vi "HeartBeatDetectOffline2BreathingSpectra.vi"() -> ()   [LabVIEW 2014, in "Phonocardiography.lvlib"]
uses:
  Phonocardiography.lvlib
  <vilib>/Waveform/WDTOps.llb/WDT Index Channel DBL.vi
  <vilib>/Waveform/WDTOps.llb/WDT Get Waveform Time Array DBL.vi
  <vilib>/measure/NI_MABase.lvlib
  <vilib>/gmath/NI_Gmath.lvlib
panel:
  out "RR intervals spectra avg":T1(graph)
  in  "Length [s]":dbl=120.0
  in  "Input files":path[](array[path])=[path "C:/Users/Tamas/Documents/Projektek/Szívhang/Felvételek cikkhez/breath_3_1.wav", path "C:/Users/Tamas/Documents/Projektek/Szívhang/Felvételek cikkhez/breath_3_2.wav", path "C:/Users/Tamas/Documents/Projektek/Szívhang/Felvételek cikkhez/breath_3_3.wav", path "C:/Users/Tamas/Documents/Projektek/Szívhang/Felvételek cikkhez/breath_3_4.wav", path "C:/Users/Tamas/Documents/Projektek/Szívhang/Felvételek cikkhez/breath_3_5.wav"]
  out "RR intervals Spectra":T2(graph)
  in  "Remove\nEctopic Beats":bool=TRUE
  out "pNN50 [%]":dbl=21.232876712328768 format="%.1f"
  out "rMSSD  [ms] 2":dbl=68.85967760569123
  out "sdRR [ms]":dbl=81.8447364744125
  out "Mean RR [ms]":dbl=843.4299467994049 format="%_1f"
  out "Mean heart rate [BPM]":dbl=71.13809537790807 format="%#.1g"
  in  "Negate":bool
  out "Heart rate":T3(graph)=[{"X [s]"=[1.0717460317460312, 1.80517006802721, 2.5313378684807244, 3.290975056689341, 4.021224489795917, 4.70439909297052, 5.478639455782311, 6.424126984126981, 7.393197278911561, 7.796190476190473, 8.327437641723353, 8.847437641723353, 9.405170068027207, 9.964353741496595, 10.772154195011334, 11.603537414965981, 12.395011337868475, 13.184852607709745, 14.145306122448973, 15.155192743764166, 16.14068027210884, 17.033469387755094, 17.822131519274368, 18.64335600907029, 19.487619047619038, 20.375328798185933, 21.22839002267573, 22.09015873015872, 23.05795918367346, 24.05832199546484, 24.99410430839001, 25.799637188208607, 26.6073469387755, 27.47473922902493, 28.39437641723355, 29.231383219954637, 29.97877551020407, 30.762539682539668, 31.684172335600895, 32.67800453514738, 33.57396825396824, 34.4517006802721, 35.36925170068026, 36.28861678004534, 37.15555555555554, 37.95655328798184, 38.77551020408161, 39.65396825396824, 40.55764172335599, 41.41306122448978, 42.231564625850325, 43.0978684807256, 43.9931065759637, 44.85678004535146, 45.67555555555553, 46.53306122448978, 47.4449886621315, 48.34476190476188, 49.17569160997731, 49.996462585033996, 50.84081632653059, 51.72117913832197, 52.59909297052152, 53.41514739229023, 54.19619047619045, 55.033197278911544, 55.98503401360542, 56.90684807256233, 57.75981859410428, 58.61931972789113, 59.50086167800451, 60.36961451247163, 61.17061224489793, 61.92444444444442, 62.72108843537412, 63.64117913832197, 64.58993197278909, 65.45814058956913, 66.26476190476188, 67.12761904761902, 67.99945578231289, 68.84235827664396, 69.60662131519271, 70.34802721088433, 71.14340136054419, 72.01424036281176, 72.89895691609975, 73.7321541950113, 74.63265306122446, 75.49950113378682, 76.35229024943307, 77.16163265306119, 77.9244444444444, 78.7406802721088, 79.62376417233557, 80.51482993197276, 81.34285714285711, 82.16371882086165, 82.98585034013603, 83.80099773242627, 84.58294784580495, 85.30902494331062, 86.04371882086164, 86.8790929705215, 87.71265306122446, 88.51310657596368, 89.29442176870745, 90.11845804988658, 91.04770975056685, 91.951746031746, 92.83129251700676, 93.60943310657592, 94.33342403628114, 95.11464852607706, 96.10811791383216, 97.0424489795918, 97.87301587301583, 98.73560090702944, 99.6119727891156, 100.47990929705212, 101.28988662131515, 102.05941043083895, 102.92235827664395, 103.86539682539679, 104.79102040816322, 105.62947845804985, 106.49442176870744, 107.41741496598635, 108.33024943310653, 109.14539682539677, 109.91655328798181, 110.7006802721088, 111.55909297052149, 112.48725623582762, 113.36698412698408, 114.20988662131515, 115.1309750566893, 116.04380952380947, 116.96145124716548, 117.8107936507936, 118.61242630385482, 119.44879818594099, 120.3123809523809, 121.14938775510198, 121.9503854875283, 122.88353741496593, 123.8236734693877], "Heart Rate [BPM]"=[70.17078604009762, 81.80806331931737, 82.62553085186114, 78.98507462686567, 82.1637063718793, 87.82527881040896, 77.49531396438616, 63.4593246354567, 61.9150131037065, 76.9022492495641, 112.94177906778204, 115.38461538461549, 107.57846804358446, 107.2992700729927, 74.27576914439706, 72.16888500981902, 75.80793032317217, 75.96463022508034, 62.47048824251586, 59.41261002335189, 60.88357109986189, 67.20512039012517, 76.07820586543993, 73.06163021868771, 71.06789858186532, 67.5896597527331, 70.33492822966507, 69.62425007893924, 61.996251171508796, 59.978239187596536, 64.11747601046817, 74.48485530908663, 74.28411005053344, 69.17285370699592, 65.24312062333553, 71.68400520156047, 80.27912621359225, 76.55363962504369, 65.1018600531442, 60.37236469836633, 66.96699736788844, 68.35796217836082, 65.39145907473319, 65.26243093922655, 69.20903954802297, 74.90657909636512, 73.26392734522106, 68.30149716055729, 66.39566395663958, 70.14102428162433, 73.30452127659571, 69.25976337556331, 67.02127659574438, 69.4706994328922, 73.28015952143613, 69.97038290670581, 65.79470857370208, 66.6834677419358, 72.20827420587224, 73.10200022101891, 71.06026426039328, 68.15371934885671, 68.34383717326173, 73.5245081693894, 76.82034606898198, 71.68400520156017, 63.03602058319041, 65.08904850929875, 70.34240748617624, 69.80793583790614, 68.0625578763246, 69.06452286489902, 74.90657909636512, 79.59331007099007, 75.31595126949817, 65.21096214511041, 63.240917782026656, 69.10781445883887, 74.38434723940055, 69.53642384106003, 68.82022471910156, 71.18261056709309, 78.50700213624546, 80.92733056031278, 75.43619568936026, 68.89907301322785, 67.81833094115196, 72.01175702155534, 66.62973408541474, 69.21628125980924, 70.35737077217718, 74.13425977810115, 78.65636147443578, 73.50816757417483, 67.94371405094435, 67.33509771986985, 72.46138678935228, 73.09392265193387, 72.98102383053818, 73.60632024034778, 76.73123767544372, 82.63585259213028, 81.66666666666627, 71.82410423452838, 71.98041349292603, 74.95750708215405, 76.7935918272568, 72.81232801320907, 64.5680819912155, 66.36901775860288, 68.21697432195603, 77.10688891479184, 82.87396642445408, 76.80250783699069, 60.39441248972906, 64.21706630424238, 72.23981653379944, 69.5583596214511, 68.46408611053663, 69.12948061448333, 74.07614781635012, 77.97029702970353, 69.5291149884375, 63.62412234298329, 64.82116609505185, 71.55993076590184, 69.36870805369146, 65.00589622641498, 65.72933227345021, 73.60632024034778, 77.80522230063454, 76.5182186234817, 69.8964497041425, 64.64379947229533, 68.20290751623874, 71.18261056709309, 65.14032496307271, 65.72933227345021, 65.38499555204083, 70.64288765484868, 74.84725050916548, 71.73842316451567, 69.47799600882185, 71.68400520156138, 74.90657909636447, 64.29821150855413, 63.82054992764095]}, {"X [s]"=array[1368064 elements], "Heart Rate [BPM]"=array[1368064 elements]}]
  out "Heart beats":cluster{"Peaks X":dbl[], "Peaks Y":dbl[]}[](graph)=[{"Peaks X"=array[1368064 elements], "Peaks Y"=array[1368064 elements]}, {"Peaks X"=[0.21668934240362803, 1.0717460317460312, 1.80517006802721, 2.5313378684807244, 3.290975056689341, 4.021224489795917, 4.70439909297052, 5.478639455782311, 6.424126984126981, 7.393197278911561, 7.796190476190473, 8.327437641723353, 8.847437641723353, 9.405170068027207, 9.964353741496595, 10.772154195011334, 11.603537414965981, 12.395011337868475, 13.184852607709745, 14.145306122448973, 15.155192743764166, 16.14068027210884, 17.033469387755094, 17.822131519274368, 18.64335600907029, 19.487619047619038, 20.375328798185933, 21.22839002267573, 22.09015873015872, 23.05795918367346, 24.05832199546484, 24.99410430839001, 25.799637188208607, 26.6073469387755, 27.47473922902493, 28.39437641723355, 29.231383219954637, 29.97877551020407, 30.762539682539668, 31.684172335600895, 32.67800453514738, 33.57396825396824, 34.4517006802721, 35.36925170068026, 36.28861678004534, 37.15555555555554, 37.95655328798184, 38.77551020408161, 39.65396825396824, 40.55764172335599, 41.41306122448978, 42.231564625850325, 43.0978684807256, 43.9931065759637, 44.85678004535146, 45.67555555555553, 46.53306122448978, 47.4449886621315, 48.34476190476188, 49.17569160997731, 49.996462585033996, 50.84081632653059, 51.72117913832197, 52.59909297052152, 53.41514739229023, 54.19619047619045, 55.033197278911544, 55.98503401360542, 56.90684807256233, 57.75981859410428, 58.61931972789113, 59.50086167800451, 60.36961451247163, 61.17061224489793, 61.92444444444442, 62.72108843537412, 63.64117913832197, 64.58993197278909, 65.45814058956913, 66.26476190476188, 67.12761904761902, 67.99945578231289, 68.84235827664396, 69.60662131519271, 70.34802721088433, 71.14340136054419, 72.01424036281176, 72.89895691609975, 73.7321541950113, 74.63265306122446, 75.49950113378682, 76.35229024943307, 77.16163265306119, 77.9244444444444, 78.7406802721088, 79.62376417233557, 80.51482993197276, 81.34285714285711, 82.16371882086165, 82.98585034013603, 83.80099773242627, 84.58294784580495, 85.30902494331062, 86.04371882086164, 86.8790929705215, 87.71265306122446, 88.51310657596368, 89.29442176870745, 90.11845804988658, 91.04770975056685, 91.951746031746, 92.83129251700676, 93.60943310657592, 94.33342403628114, 95.11464852607706, 96.10811791383216, 97.0424489795918, 97.87301587301583, 98.73560090702944, 99.6119727891156, 100.47990929705212, 101.28988662131515, 102.05941043083895, 102.92235827664395, 103.86539682539679, 104.79102040816322, 105.62947845804985, 106.49442176870744, 107.41741496598635, 108.33024943310653, 109.14539682539677, 109.91655328798181, 110.7006802721088, 111.55909297052149, 112.48725623582762, 113.36698412698408, 114.20988662131515, 115.1309750566893, 116.04380952380947, 116.96145124716548, 117.8107936507936, 118.61242630385482, 119.44879818594099, 120.3123809523809, 121.14938775510198, 121.9503854875283, 122.88353741496593, 123.8236734693877], "Peaks Y"=[0.201629638671875, 0.192962646484375, 0.213836669921875, 0.209014892578125, 0.205413818359375, 0.18658447265625, 0.20831298828125, 0.272430419921875, 0.238372802734375, 0.219329833984375, 0.125732421875, 0.18994140625, 0.128082275390625, 0.09893798828125, 0.183624267578125, 0.169097900390625, 0.19970703125, 0.200042724609375, 0.220733642578125, 0.21014404296875, 0.22100830078125, 0.17681884765625, 0.207855224609375, 0.21734619140625, 0.164459228515625, 0.166290283203125, 0.189208984375, 0.193267822265625, 0.1942138671875, 0.163330078125, 0.218475341796875, 0.165557861328125, 0.157012939453125, 0.152130126953125, 0.137481689453125, 0.184234619140625, 0.1441650390625, 0.166717529296875, 0.128570556640625, 0.168548583984375, 0.168731689453125, 0.149444580078125, 0.14691162109375, 0.1910400390625, 0.15167236328125, 0.13525390625, 0.175018310546875, 0.123992919921875, 0.168548583984375, 0.15008544921875, 0.141387939453125, 0.139434814453125, 0.14385986328125, 0.151214599609375, 0.151275634765625, 0.166107177734375, 0.11834716796875, 0.174407958984375, 0.137786865234375, 0.151580810546875, 0.13751220703125, 0.139801025390625, 0.17926025390625, 0.14227294921875, 0.141571044921875, 0.14837646484375, 0.13397216796875, 0.186920166015625, 0.125518798828125, 0.149078369140625, 0.15155029296875, 0.15460205078125, 0.1619873046875, 0.116912841796875, 0.1724853515625, 0.12261962890625, 0.166290283203125, 0.150177001953125, 0.148468017578125, 0.18017578125, 0.120941162109375, 0.151336669921875, 0.158203125, 0.1790771484375, 0.137786865234375, 0.156158447265625, 0.166778564453125, 0.147857666015625, 0.17822265625, 0.1409912109375, 0.143402099609375, 0.159912109375, 0.14312744140625, 0.17120361328125, 0.1217041015625, 0.15777587890625, 0.148040771484375, 0.17626953125, 0.146087646484375, 0.119842529296875, 0.1455078125, 0.134796142578125, 0.153167724609375, 0.155242919921875, 0.149688720703125, 0.152496337890625, 0.16204833984375, 0.188507080078125, 0.146392822265625, 0.1685791015625, 0.17132568359375, 0.12103271484375, 0.1685791015625, 0.154754638671875, 0.14630126953125, 0.1690673828125, 0.1383056640625, 0.16705322265625, 0.126739501953125, 0.16619873046875, 0.13958740234375, 0.1534423828125, 0.144744873046875, 0.1336669921875, 0.157562255859375, 0.1373291015625, 0.16473388671875, 0.1514892578125, 0.15313720703125, 0.13812255859375, 0.1527099609375, 0.17401123046875, 0.150604248046875, 0.1429443359375, 0.15435791015625, 0.147735595703125, 0.1685791015625, 0.146759033203125, 0.157257080078125, 0.150054931640625, 0.152862548828125, 0.13958740234375, 0.13262939453125, 0.1474609375, 0.147857666015625, 0.157257080078125, 0.140716552734375, 0.164642333984375]}]
  in  "Max time to peak\nfrom threshold (ms)":dbl=150.0
  in  "Threshold mult 2":dbl=0.4 min=-1.0 max=1.0 step=0.05
  in  "Min time between\nbeats (ms)":dbl=450.0
  in  "width (threshold) 2":i32=3
  in  "Breathing freq \n[1/min]":dbl=15.0
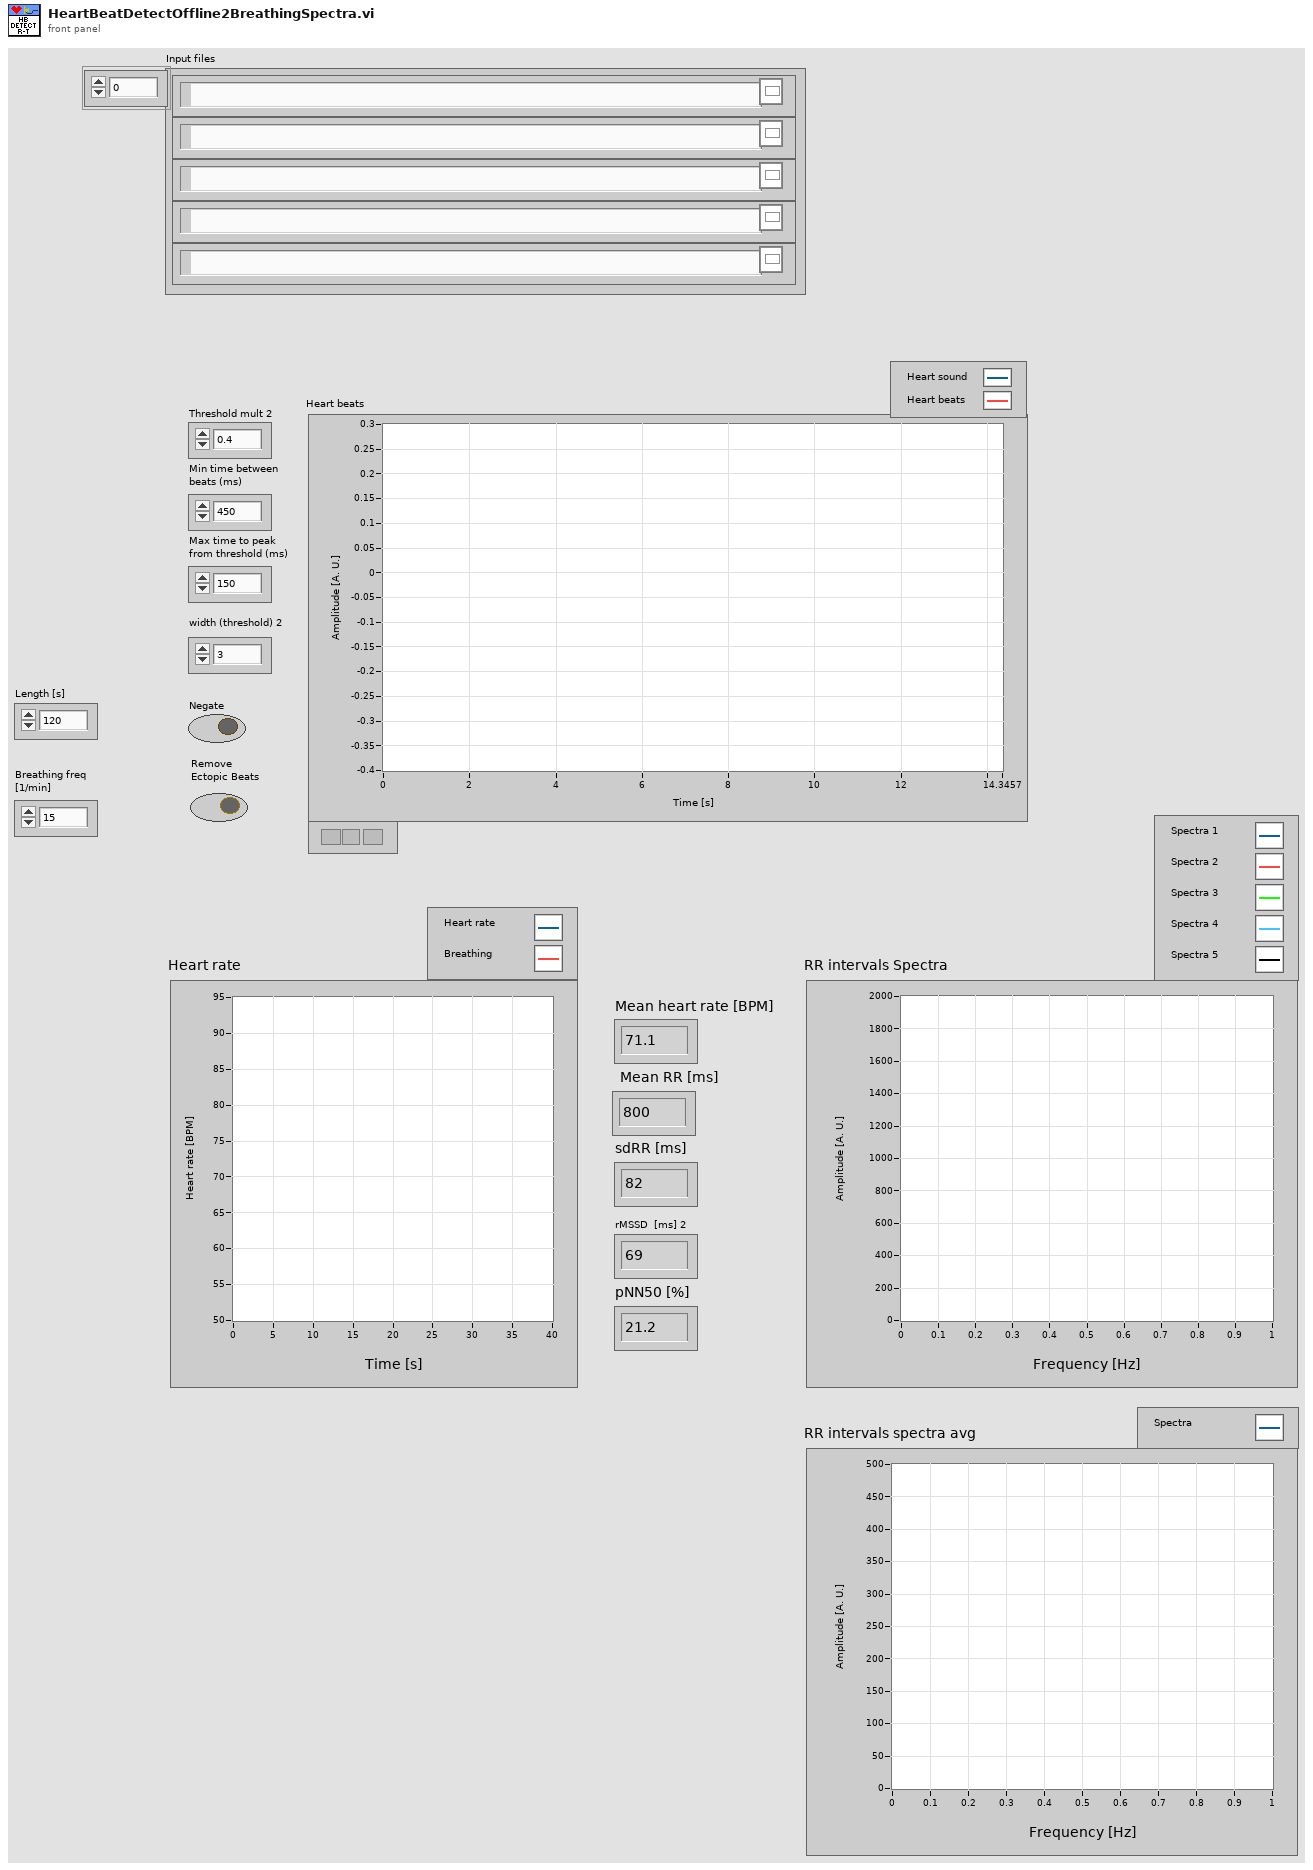
[diagram p1: front panel]
types:
  T1 = cluster{"Power Spectrum FFT {X} Frequency":dbl[], dbl[]}
  T2 = cluster{"Power Spectrum FFT {X} Frequency":dbl[], "Power Spectrum FFT {X}":dbl[]}[]
  T3 = cluster{"X [s]":dbl[], "Heart Rate [BPM]":dbl[]}[]
  T4 = typedef "LVCursorListTypeDef.ctl" = cluster{"Name":string, "Color":u32, "Style":u8, "Point Style":u8, "Name Visible":bool, "Allow Drag":bool, "Cursor Mode":u32, "Plot":i32, "Index":i32, "Position":cluster{"X":dbl, "Y":dbl}, "X Scale":u32, "Y Scale":u32, "Watch Plots":i32[], "Watch All Plots":bool, "Plot Area":i32, "Label Offset":cluster{"X":dbl, "Y":dbl}}[]
  T5 = cluster{"Name":string, "Color":u32, "Style":u8, "Point Style":u8, "Name Visible":bool, "Allow Drag":bool, "Cursor Mode":u32, "Plot":i32, "Index":i32, "Position":cluster{"X":dbl, "Y":dbl}, "X Scale":u32, "Y Scale":u32, "Watch Plots":i32[], "Watch All Plots":bool, "Plot Area":i32, "Label Offset":cluster{"X":dbl, "Y":dbl}}
  T6 = cluster{"Name":string, "Color":u32, "Style":u8, "Point Style":u8, "Name Visible":bool, "Allow Drag":bool, "Cursor Mode":u32, "Plot":i32, "Index":i32, "Position":cluster{"X":dbl, "Y":dbl}, "X Scale":u32, "Y Scale":u32, "Watch Plots":i32[], "Watch All Plots":bool, "Plot Area":i32, "Label Offset":cluster{"X":dbl, "Y":dbl}}[]
  T7 = cluster{"Power Spectrum FFT {X} Frequency":dbl[], "Power Spectrum FFT {X}":dbl[]}
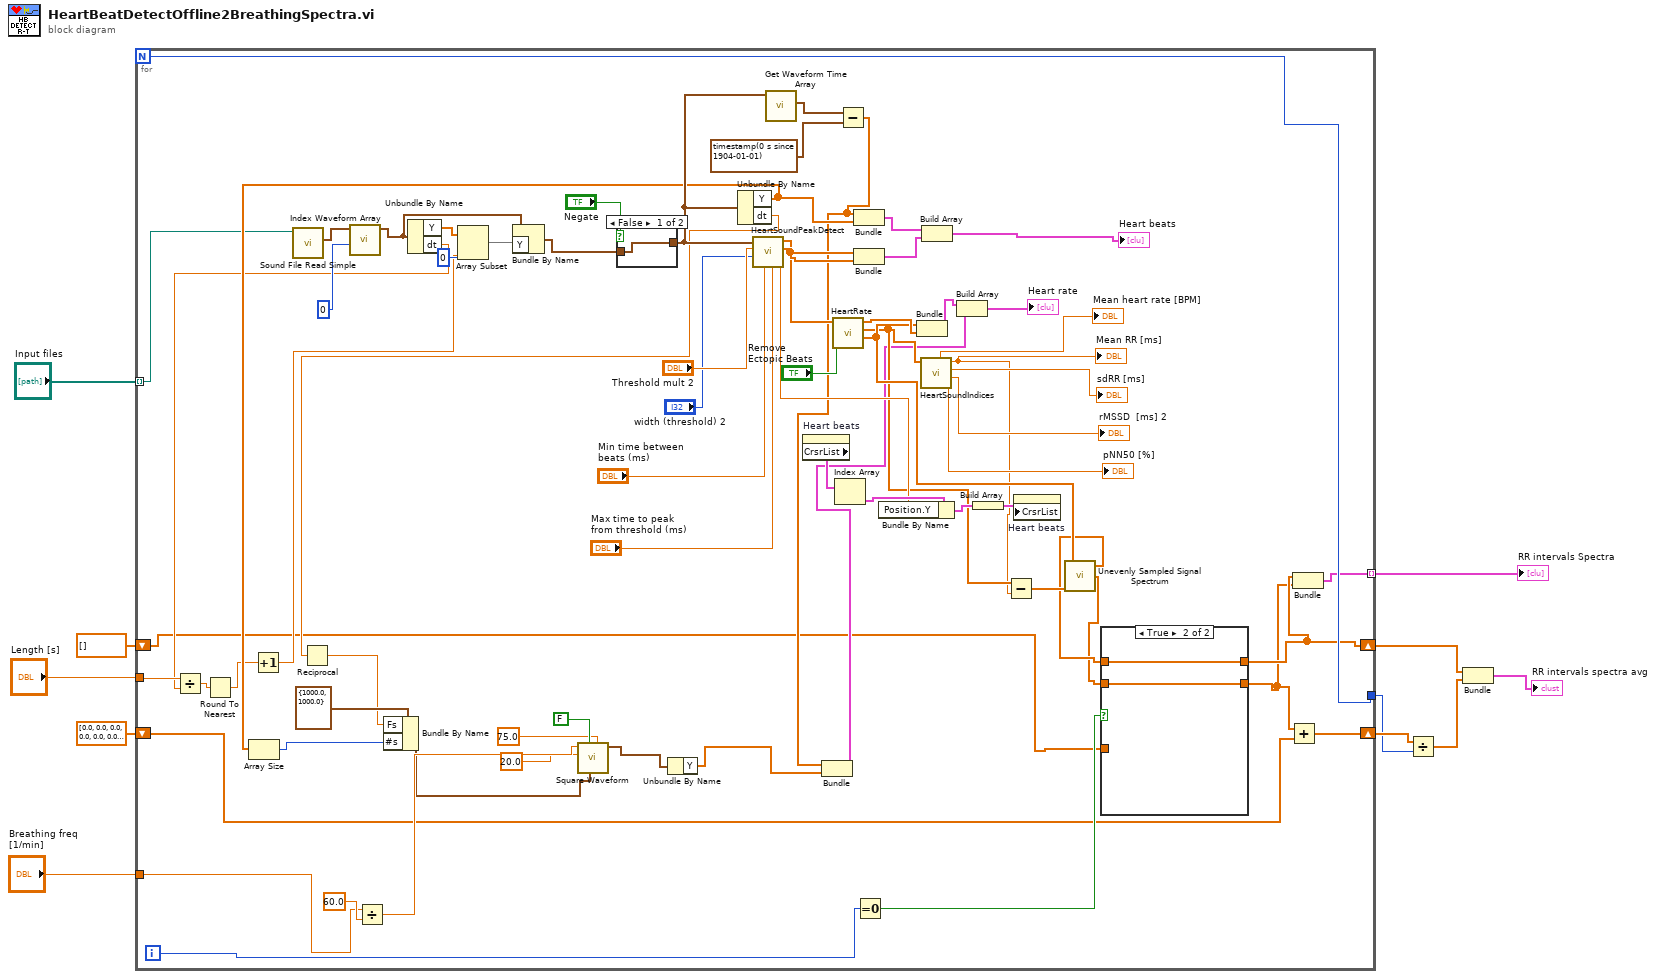
[diagram p0: block diagram]
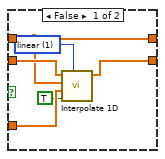
[diagram p2: hidden frame]
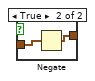
[diagram p3: hidden frame]
diagram:
  n1 = for {
    N -> [w16]
    tunnel: "Breathing freq \n[1/min]" -> [w77]
    tunnel: "Input files" -> [w34] mode=indexing
    tunnel: "Length [s]" -> [w33]
    shift-right: [w15] -> w3
    shift-left: dbl[] [] ("Power Spectrum FFT {X} Frequency") -> [w18]
    shift-right: [w17] -> w6
    shift-left: dbl[] [0.0, 0.0, 0.0, 0.0, 0.0, 0.0, 0.0, 0.0, 0.0, 0.0, 0.0, 0.0, 0.0, 0.0, 0.0, 0.0, 0.0, 0.0, 0.0, 0.0, 0.0, 0.0, 0.0, 0.0, 0.0, 0.0, 0.0, 0.0, 0.0, 0.0, 0.0, 0.0, 0.0, 0.0, 0.0, 0.0, 0.0, 0.0, 0.0, 0.0, 0.0, 0.0, 0.0, 0.0, 0.0, 0.0, 0.0, 0.0, 0.0, 0.0, 0.0, 0.0, 0.0, 0.0, 0.0, 0.0, 0.0, 0.0, 0.0, 0.0, 0.0, 0.0, 0.0, 0.0, 0.0, 0.0, 0.0, 0.0, 0.0, 0.0, 0.0, 0.0, 0.0, 0.0, 0.0, 0.0, 0.0, 0.0, 0.0, 0.0, 0.0, 0.0, 0.0, 0.0, 0.0, 0.0, 0.0, 0.0, 0.0, 0.0, 0.0, 0.0, 0.0, 0.0, 0.0, 0.0, 0.0, 0.0, 0.0, 0.0, 0.0, 0.0, 0.0, 0.0, 0.0, 0.0, 0.0, 0.0, 0.0, 0.0, 0.0, 0.0, 0.0, 0.0, 0.0, 0.0, 0.0, 0.0, 0.0, 0.0, 0.0, 0.0, 0.0, 0.0, 0.0, 0.0, 0.0, 0.0, 0.0, 0.0, 0.0, 0.0, 0.0, 0.0, 0.0, 0.0, 0.0, 0.0, 0.0, 0.0, 0.0, 0.0, 0.0, 0.0, 0.0, 0.0, 0.0, 0.0, 0.0, 0.0, 0.0] -> [w12]
    tunnel: [w16] -> w5
    tunnel: [w14] -> w4 mode=indexing
    i -> [w20]
    n2 = call <vilib>:"Sound File Read Simple.vi"("path"=w34) -> ("data"=w76:waveform(dbl)[])  [unwired: 7 in, 3 out]
    n3 = call-poly <vilib>:"Index Waveform Array.vi"("index"=0, "waveform array"=w76) -> ("waveform"=w28:waveform(dbl))  [unwired: 8 in, 1 out]
    n4 = Divide(x=w77, y=60.0) -> (x/y=w80:dbl)
    n5 = Unbundle By Name(w28) -> ("Y"=w27:dbl[], "dt"=w29:dbl)
    n6 = Divide(x=w33, y=w29) -> (x/y=w31:dbl)
    n7 = Round To Nearest(number=w31) -> (nearest integer value=w30:dbl)
    n8 = Increment(x=w30) -> (x+1=w23:dbl)
    n9 = Array Subset(array=w27, index=0, length=w23) -> (w26:dbl[])
    n10 = Bundle By Name(cluster=w28, "Y"=w26) -> (w25:waveform(dbl))
    n11 = case shown="False" "Negate" {
      tunnel: w25 -> [w90 w92]
      tunnel: [w90 w91] -> w57
      frame False {
      }
      frame True {
        n12 = Negate(x=w92) -> (-x=w91:waveform(dbl))
      }
    }
    n13 = Unbundle By Name(w57) -> ("Y"=w43:dbl[], "dt"=w32:dbl)
    n14 = Array Size(array=w43) -> (size(s)=w42:i32)
    n15 = Reciprocal(x=w32) -> (1/x=w37:dbl)
    n16 = Bundle By Name(cluster=cluster{"Fs":dbl, "#s":dbl} {"Fs"=1000.0, "#s"=1000.0} ("sampling info"), "Fs"=w37, "#s"=w42) -> (w78:cluster{"Fs":dbl, "#s":dbl})
    n17 = call <vilib>:"Square Waveform.vi"("offset"=75.0 ("amplitude"), "sampling info"=w78, "reset signal"=FALSE, "amplitude"=20.0, "frequency"=w80) -> ("signal out"=w45:waveform(dbl))  [unwired: 5 in, 1 out]
    n18 = Unbundle By Name(w45) -> ("Y"=w36:dbl[])
    n19 = call "HeartSoundPeakDetect.vi"("Max time to peak\nfrom threshold (ms)"="Max time to peak\nfrom threshold (ms)", "Min time between\nbeats (ms)"="Min time between\nbeats (ms)", "width (threshold)"="width (threshold) 2", "Threshold multiplier"="Threshold mult 2", "Sound"=w57) -> ("Threshold"=w58:dbl, "Peaks Y"=w70:dbl[], "Peaks X"=w67:dbl[])  [unwired: 4 in]
    n20 = call-poly <vilib>:"Get Waveform Time Array.vi"("waveform in"=w57) -> ("X array"=w65:timestamp[])  [unwired: 9 in, 1 out]
    n21 = property on="Heart beats" class="XYGraph (strict)"() -> ("CrsrList"=w60:T4)  [unwired: 2 in, 2 out]
    n22 = call "HeartRate.vi"("Remove Ectopic?"="Remove\nEctopic Beats", "Peaks X in"=w67) -> ("X [s]"=w50:dbl[], "RR intervals [ms]"=w48:dbl[], "Heart Rate [BPM]"=w66:dbl[])  [unwired: 7 in]
    n23 = Index Array(array=w60) -> (element=w62:T5)  [unwired: 1 in]
    n24 = Subtract(x=w65, y=timestamp(0 s since 1904-01-01) ("Xo")) -> (x-y=w41:dbl[])
    n25 = Bundle(w41, "Y"=w36) -> (w39:cluster{dbl[], "Y":dbl[]})  [unwired: 1 in]
    n26 = Bundle(w41, "Y"=w43) -> (w69:cluster{dbl[], "Y":dbl[]})  [unwired: 1 in]
    n27 = Bundle("Peaks X"=w67, "Peaks Y"=w70) -> (w68:cluster{"Peaks X":dbl[], "Peaks Y":dbl[]})  [unwired: 1 in]
    n28 = Equal To 0?(x=w20) -> (x = 0?=w19:bool)
    n29 = Bundle By Name(cluster=w62, "Position.Y"=w58) -> (w61:T5)
    n30 = Bundle("X [s]"=w50, "Heart Rate [BPM]"=w66) -> (w40:cluster{"X [s]":dbl[], "Heart Rate [BPM]":dbl[]})  [unwired: 1 in]
    n31 = call "HeartSoundIndices.vi"("RR intervals [ms]"=w48) -> ("pNN50 [%]"=→"pNN50 [%]":dbl, "rMSSD  [ms]"=→"rMSSD  [ms] 2":dbl, "sdRR [ms]"=→"sdRR [ms]":dbl, "Mean RR [ms]"=w47:dbl, "Mean heart rate [BPM]"=→"Mean heart rate [BPM]":dbl)  [unwired: 6 in]
    "Mean RR [ms]" <- w47
    n32 = Build Array(w69, w68) -> (→"Heart beats":cluster{"Peaks X":dbl[], "Peaks Y":dbl[]}[])
    n33 = Build Array(w40, w39) -> (→"Heart rate":cluster{"X [s]":dbl[], "Y":dbl[]}[])
    n34 = Build Array(w61) -> (w59:T6)
    n35 = Subtract(x=w48, y=w47) -> (x-y=w49:dbl[])
    n36 = property on="Heart beats" class="XYGraph (strict)"("CrsrList"=w59) -> ()  [unwired: 2 in, 2 out]
    n37 = call <vilib>:"Unevenly Sampled Signal Spectrum.vi"("XTime"=w50, "X"=w49) -> ("Power Spectrum FFT {X} Frequency"=w22:dbl[], "Power Spectrum FFT {X}"=w21:dbl[])  [unwired: 1 out]
    n38 = case shown="True" w19 {
      tunnel: w22 -> [w86 w89]
      tunnel: w21 -> [w87 w88]
      tunnel: [w86 w89] -> w15
      tunnel: [w83 w88] -> w13
      tunnel: w18 -> [w85 _]
      frame False {
        w82 = 1 items=["nearest", "linear", "spline", "cubic Hermite", "Lagrange"] ("method")
        n39 = call <vilib>:"Interpolate 1D.vi"("method"=w82, "X is monotonic"=TRUE, "xi"=w85, "X"=w86, "Y"=w87) -> ("yi"=w83:dbl[])  [unwired: 4 in, 2 out]
      }
      frame True {
      }
    }
    n40 = Add(x=w13, y=w12) -> (x+y=w17:dbl[])
    n41 = Bundle("Power Spectrum FFT {X} Frequency"=w15, "Power Spectrum FFT {X}"=w13) -> (w14:T7)  [unwired: 1 in]
  }
  "RR intervals Spectra" <- w4
  n42 = Divide(x=w6, y=w5) -> (x/y=w2:dbl[])
  n43 = Bundle("Power Spectrum FFT {X} Frequency"=w3, w2) -> (→"RR intervals spectra avg":T1)  [unwired: 1 in]
